vi "Alyssa_GlueFatLines.vi"(5 "Image Feed":T6=refnum, 7 "Template Path":path=path "C:/Users/Aerotech/Documents/BNL_ThermomechanicalStave/Utils/ConfigurationFiles_and_Templates/1_ModulePlacement", 8 "error in":errorcluster, 9 "um/pix resolution":dbl=1.58, 10 "Module corner coordinates":T2={"X [mm]"=-59.42477770816987, "Y [mm]"=4.341763392096446, "Z [mm] "=36.00000100000001}, 11 "XYZ Stage Control":refnum<k24>) -> (0 "error out":errorcluster={"status"=FALSE, "code"=1073676418, "source"="VISA Close in Alyssa_GlueFatLines.vi"}, 3 "XYZ .NET Refnum out":refnum<k24>)   [LabVIEW 2016]
uses:
  C:/Users/Aerotech/Documents/BNLStaveAssembly-blueprint/Bin/Aerotech.A3200.dll
  BNLStaveAssembly-blueprint/Bin/Aerotech.A3200.dll
  <vilib>/vision/Image Controls.llb/IMAQ Image.ctl
  <vilib>/LabVIEW Interface for Arduino/Type Defs/Arduino Resource.ctl
  <vilib>/LabVIEW Interface for Arduino/Type Defs/Board Type.ctl
  <vilib>/LabVIEW Interface for Arduino/Type Defs/Pin Mode.ctl
  <vilib>/Analysis/coordinate.llb/2D Cartesian Coordinate Rotation (Scalar).vi
  <vilib>/LabVIEW Interface for Arduino/LabVIEW Interface for Arduino.lvlib
  <vilib>/Analysis/NI_AALPro.lvlib
panel:
  in  "?":T1(tab)
  in  "Axis speeds (mm/s)":T3={"vX [mm]"=40.0, "vY [mm]"=40.0, "vZ [mm] "=40.0}
  in  "Home?":bool
  in  "Lowest Z Position":dbl=38.0
  out "Arduino Resource":T4={"VISA resource"="GlueCTRL", "Board Type"=enum."Uno", "Connection Type"=enum."USB / Serial", "Bytes Per Packet (15)"=15}
  in  "Digital I/O Pin":u8=7
  in  "Testing?":bool
  out "Difference camera/syringe in X":dbl=-133.03368290747076
  out "Difference camera/syringe in y":dbl=-2.170984960815403
  in  "Path to save collected images":path=path "C:/Users/Aerotech/cernbox/BNL/Stave Assembly Records/2017-06-12/3"
  in  "Estimate distance y":dbl
  in  "Estimate distance x":dbl=130.0
  in  "Lowest Z position Calibration":dbl=17.0
  in  "How many lines (actual x2)":i32=7
  in  "y dist (mm)":dbl=4.5
  out "bottom line speed":cluster{dbl, dbl, dbl}={32.78688524590164, 32.78688524590164, 32.78688524590164}
  out "mid line speed":cluster{dbl, dbl, dbl}={21.85792349726776, 21.85792349726776, 21.85792349726776}
  in  "Axial?":enum32{"Axial", "Right Stereo", "Left Stereo"}(radio)
  in  "glue time":dbl=1.83 format="%#_13g"
  out "top right speed":cluster{dbl, dbl, dbl}={5.46448087431694, 5.46448087431694, 5.46448087431694}
  out "top left speed":cluster{dbl, dbl, dbl}={21.85792349726776, 21.85792349726776, 21.85792349726776}
  out "Final Position":T7={"Final X"=-59.424942872475754, "Final Y"=8.342749448838399, "Final Z"=36.000300999844}
  out "Module Start":T7={"Final X"=-59.42477770816987, "Final Y"=4.341763392096446, "Final Z"=36.00000100000001}
  # "Overview: This takes a pattern of zeroes/ones (.csv file) as well as the start coordinates of the top left corner of a module and places dots of glue  \nRequirements: NI Arduino dependencies\nInstructions: Select a .csv file (ones indicate regions for glue) as well as a starting coordinate (this is default to the top left corner of the module spacer). You \ncan also input axis speeds (default to maximum) and module lengths and widths (default to 90 mm) which are the widths of the module to which you want to \nplace glue. Lastly, one can choose to Home the stage here and can select the lowest position in Z. The default is that the stage moves down 2-3 mm in Z \nwhile dispensing.  The Arduino inputs are default and simply allow the LabView program to drigger the Arduino (which sends a signal to the dispenser). The \nprogram signals to dispense air- all other parameters such as length of dispensing (default: 350 millisec), pressure (default: 48 psi), and vacuum pressure \n(default: 7.8 psi) are set on the dispenser itself. The defaults are highly recommended here."
  # "Positioning Inputs"
  # "Arduino Inputs"
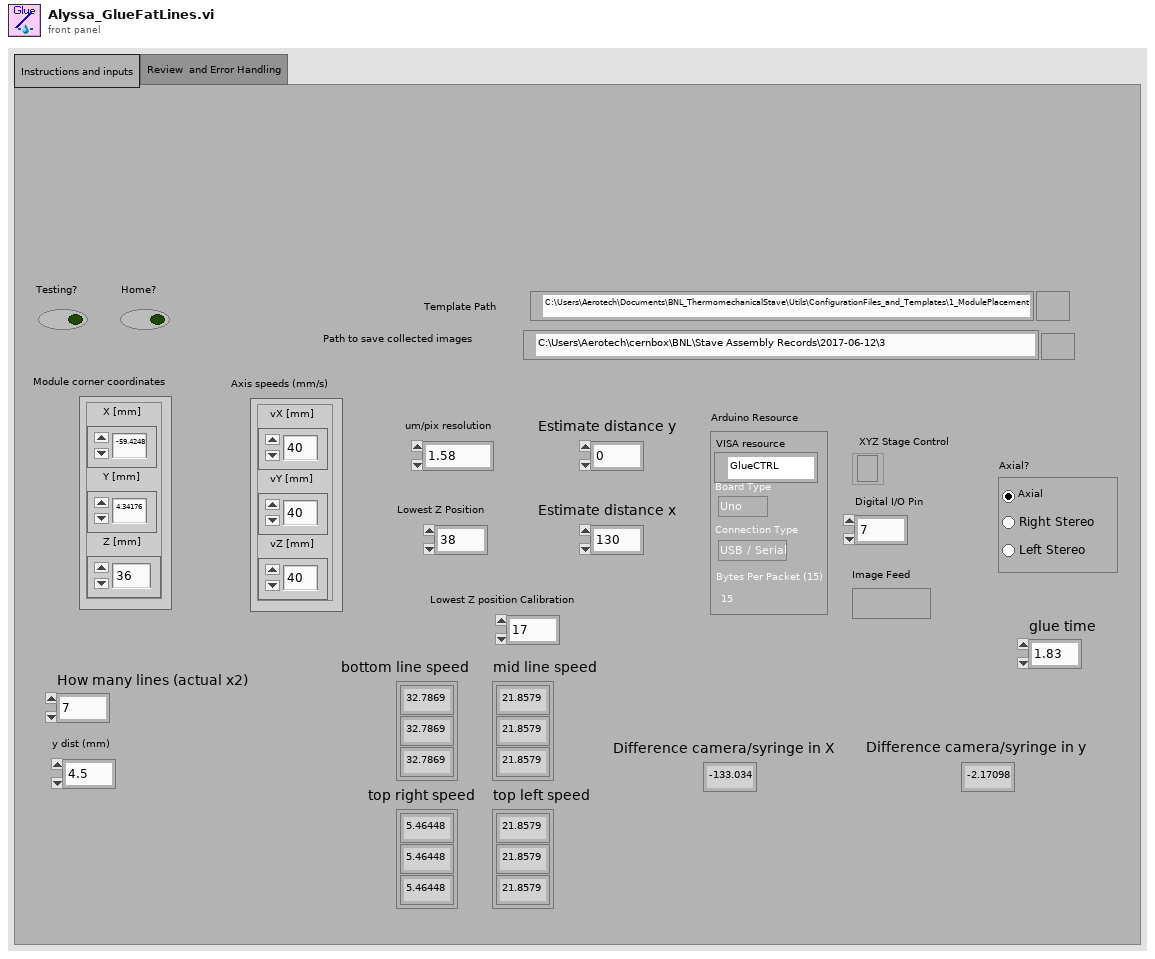
[diagram p1: front panel]
types:
  T1 = enum32{"Instructions and inputs", "Review  and Error Handling"}
  T2 = cluster{"X [mm]":dbl, "Y [mm]":dbl, "Z [mm] ":dbl}
  T3 = cluster{"vX [mm]":dbl, "vY [mm]":dbl, "vZ [mm] ":dbl}
  T4 = typedef "LabVIEW Interface for Arduino.lvlib/Arduino Resource.ctl" = cluster{"VISA resource":refnum<visa-resource-name>, "Board Type":T5, "Connection Type":enum8{"USB / Serial"}, "Bytes Per Packet (15)":u8}
  T5 = typedef "LabVIEW Interface for Arduino.lvlib/Board Type.ctl" = enum16{"Uno", "Dimuelanove w/Atmega 328", "Mega 2560"}
  T6 = typedef "IMAQ Image.ctl" = refnum<image>
  T7 = cluster{"Final X":dbl, "Final Y":dbl, "Final Z":dbl}
  T8 = typedef "LabVIEW Interface for Arduino.lvlib/Pin Mode.ctl" = enum8{"Input", "Output"}
  T9 = cluster{dbl, "Y [mm]":dbl, "Lowest Z Position":dbl}
  T10 = cluster{"Final X":dbl, "Final Y":dbl, "vZ [mm]":dbl}
  T11 = cluster{dbl, "Final Y":dbl, "Lowest Z Position":dbl}
  T12 = cluster{"Final X":dbl, "Final Y":dbl, "Z [mm] ":dbl}
  T13 = cluster{"x out":dbl, "y out":dbl, "Lowest Z Position":dbl}
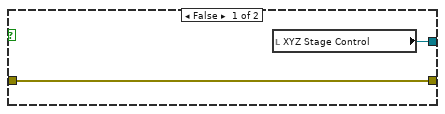
[diagram p2: hidden frame]
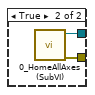
[diagram p3: hidden frame]
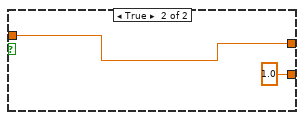
[diagram p5: hidden frame]
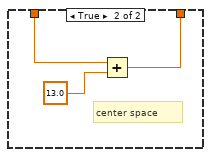
[diagram p6: hidden frame]
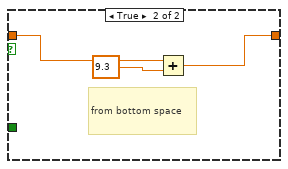
[diagram p7: hidden frame]
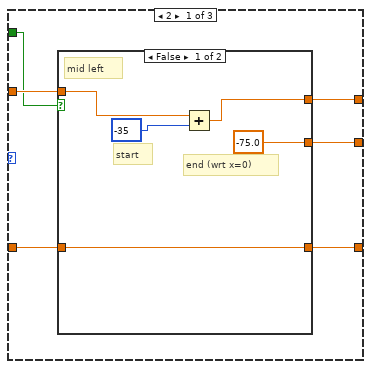
[diagram p8: hidden frame]
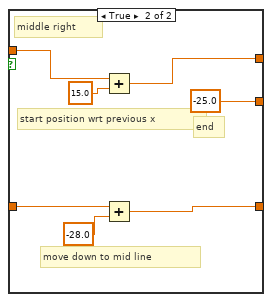
[diagram p9: hidden frame]
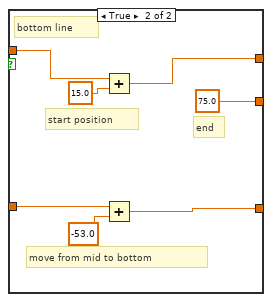
[diagram p10: hidden frame]
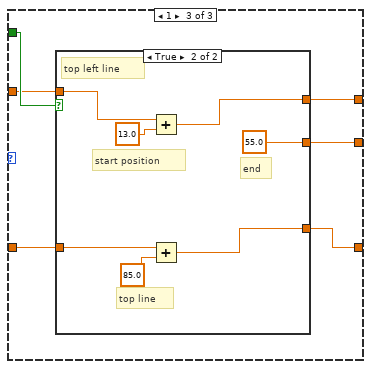
[diagram p11: hidden frame]
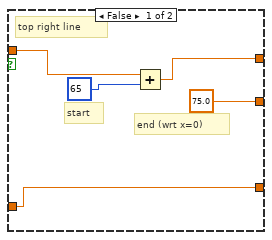
[diagram p12: hidden frame]
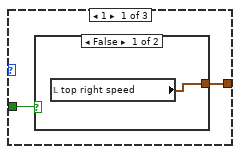
[diagram p13: hidden frame]
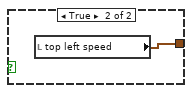
[diagram p14: hidden frame]
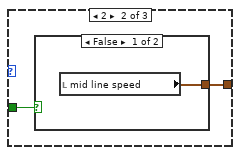
[diagram p15: hidden frame]
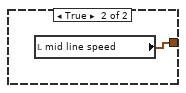
[diagram p16: hidden frame]
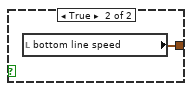
[diagram p17: hidden frame]
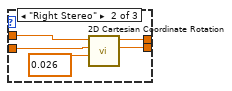
[diagram p18: hidden frame]
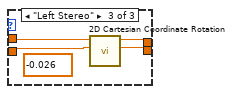
[diagram p19: hidden frame]
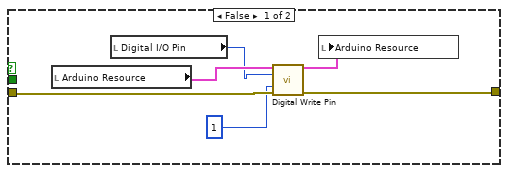
[diagram p20: hidden frame]
diagram:
  n1 = case shown="True" "Testing?" {
    tunnel: [w9 w11] -> w3
    tunnel: [w8 w10] -> w5
    tunnel: "error in" -> [w8 _]
    frame False {
      n2 = local read "XYZ Stage Control"() -> (w9:refnum<k24>)
    }
    frame True {
      n3 = case shown="False" "Home?" {
        tunnel: [w15 w21] -> w11
        tunnel: [w14 w20] -> w10
        frame False {
          w17 = string[] ["X", "Y", "Z"] ("Axes Names")
          n4 = call "Connect.vi"() -> ("error out"=w18:errorcluster, "controller"=w13:refnum<k24>)  [unwired: 10 in]
          n5 = call "EnableMultiple.vi"("error in (no error)"=w18, "axis names"=w17, "controller in"=w13) -> ("error out"=w19:errorcluster, "controller out"=w16:refnum<k24>)  [unwired: 7 in]
          n6 = call "GetCurrentXYZPosition (SubVI).vi"(".NET Refnum in - Device"=w16, "error in (no error)"=w19, "Axes Names"=w17) -> ("error out"=w14:errorcluster, ".NET Refnum out  - Device"=w15:refnum<k24>)  [unwired: 3 in, 4 out]
        }
        frame True {
          n7 = call "0_HomeAllAxes (SubVI).vi"() -> ("error out"=w20:errorcluster, "controller out"=w21:refnum<k24>)  [unwired: 8 in, 2 out]
        }
      }
    }
  }
  n8 = flat-sequence {
    tunnel: [w39] -> w7
    tunnel: w5 -> [w29]
    tunnel: w3 -> [w23]
    tunnel: [w192] -> w2
    tunnel: w7 -> [w195]
    tunnel: w2 -> [w347]
    tunnel: "Axial?" -> [w318]
    frame #0 {
      n9 = flat-sequence {
        tunnel: w29 -> [w53]
        tunnel: [w52] -> w24
        tunnel: w23 -> [w46]
        tunnel: w24 -> [w55]
        tunnel: [w54] -> w22
        tunnel: [w74] -> w26
        tunnel: w22 -> [w73]
        tunnel: w26 -> [w135]
        tunnel: [w133] -> w25
        tunnel: [w168] -> w27
        tunnel: w25 -> [w169]
        frame #0 {
          n10 = local read "Module corner coordinates"() -> (w48:T2)
          n11 = Unbundle(w48) -> ("X [mm]"=w45:dbl, "Y [mm]"=w42:dbl)  [unwired: 1 out]
          n12 = local read "Axis speeds (mm/s)"() -> (w51:T3)
          n13 = Add(x=w45, y=133.0) -> (x+y=w43:dbl)
          n14 = Bundle(w43, "Y [mm]"=w42, "Lowest Z Position"="Lowest Z Position") -> (w47:T9)  [unwired: 1 in]
          n15 = Bundle(w43, "Y [mm]"=w42, "Lowest Z Position"="Lowest Z Position") -> (w40:T9)  [unwired: 1 in]
          n16 = call "Go2XYZ (SubVI).vi"(".NET Refnum in"=w46, "Go to Coordinates"=w47, "Axis Speeds"=w51, "error in (no error)"=w53) -> (".NET Refnum out"=w50:refnum<k24>, "Final Position"=→"Final Position":T7, "error out"=w52:errorcluster)  [unwired: 7 in, 2 out]
          n17 = local write "Module corner coordinates"(w40) -> ()
          n18 = local write "XYZ Stage Control"(w50) -> ()
        }
        frame #1 {
          n19 = while {
            tunnel: w55 -> [w72]
            tunnel: [w68] -> w54
            stop <- w71 stop-if-true
            n20 = local read "Module corner coordinates"() -> (w66:T2)
            n21 = call "Lower glue mount"("error in (no error)"=w72) -> ("Move Z down"=w63:dbl, "Move Z up"=w62:dbl, "Accept current Z?"=w71:bool, "error out"=w69:errorcluster)  [unwired: 14 in, 1 out]
            n22 = local read "Lowest Z Position"() -> (w56:dbl)
            n23 = local read "Axis speeds (mm/s)"() -> (w70:T3)
            n24 = local read "XYZ Stage Control"() -> (w58:refnum<k24>)
            n25 = Add(x=w56, y=w63) -> (x+y=w60:dbl)
            n26 = Subtract(x=w60, y=w62) -> (x-y=w59:dbl)
            n27 = Unbundle(w66) -> ("X [mm]"=w65:dbl, "Y [mm]"=w64:dbl)  [unwired: 1 out]
            n28 = Bundle("X [mm]"=w65, "Y [mm]"=w64, w59) -> (w61:cluster{"X [mm]":dbl, "Y [mm]":dbl, dbl})  [unwired: 1 in]
            n29 = local write "Lowest Z Position"(w59) -> ()
            n30 = call "Go2XYZ (SubVI).vi"(".NET Refnum in"=w58, "Go to Coordinates"=w61, "Axis Speeds"=w70, "error in (no error)"=w69) -> (".NET Refnum out"=w67:refnum<k24>, "Final Position"=w57:T7, "error out"=w68:errorcluster)  [unwired: 7 in, 2 out]
            n31 = local write "XYZ Stage Control"(w67) -> ()
            n32 = local write "Final Position"(w57) -> ()
          }
        }
        frame #2 {
          n33 = call "Calibrate distance?"("error in (no error)"=w73) -> ("Calibrate distance?"=w75:bool, "error out"=w76:errorcluster)  [unwired: 16 in, 1 out]
          n34 = case shown="True" w75 {
            tunnel: w76 -> [w77 w79]
            tunnel: [w77 w80] -> w74
            frame False {
            }
            frame True {
              n35 = flat-sequence {
                tunnel: w79 -> [w82]
                tunnel: [w81] -> w78
                frame #0 {
                  n36 = local read "Final Position"() -> (w89:T7)
                  n37 = local read "Axis speeds (mm/s)"() -> (w85:T3)
                  n38 = local read "XYZ Stage Control"() -> (w84:refnum<k24>)
                  n39 = Unbundle(w89) -> ("Final X"=w87:dbl, "Final Y"=w88:dbl)  [unwired: 1 out]
                  n40 = Bundle("Final X"=w87, "Final Y"=w88, "vZ [mm]"=-20.0) -> (w91:T10)  [unwired: 1 in]
                  n41 = call "Go2XYZ (SubVI).vi"(".NET Refnum in"=w84, "Go to Coordinates"=w91, "Axis Speeds"=w85, "error in (no error)"=w82) -> (".NET Refnum out"=w83:refnum<k24>, "Final Position"=w86:T7, "error out"=w81:errorcluster)  [unwired: 7 in, 2 out]
                  n42 = local write "XYZ Stage Control"(w83) -> ()
                  n43 = local write "Final Position"(w86) -> ()
                }
              }
              n44 = while {
                tunnel: [w132] -> w80
                tunnel: w78 -> [w120]
                i -> [w117]
                stop <- w92 stop-if-true
                n45 = local read "Final Position"() -> (w94:T7)
                n46 = Unbundle(w94) -> ("Final X"=w99:dbl, "Final Y"=w97:dbl, "Final Z"=w98:dbl)
                n47 = local read "Testing?"() -> (w115:bool)
                n48 = local read "Axis speeds (mm/s)"() -> (w122:T3)
                n49 = local read "XYZ Stage Control"() -> (w118:refnum<k24>)
                n50 = Subtract(x=w97, y=220.0) -> (x-y=w95:dbl)
                n51 = Equal To 0?(x=w117) -> (x = 0?=w116:bool)
                n52 = And(x=w115, y=w116) -> (x .and. y?=w114:bool)
                n53 = Bundle("Final X"=w99, w95, "Final Z"=w98) -> (w100:cluster{"Final X":dbl, dbl, "Final Z":dbl})  [unwired: 1 in]
                n54 = call "CalibrateDistanceCameraSyringe.vi"("Path to save collected images"="Path to save collected images", "Image Feed"="Image Feed", "Off stave position"=w100, ".NET Refnum in"=w118, "Axis speeds (mm/s)"=w122, "Lowest Z Position"="Lowest Z position Calibration", "Estimate distance y"="Estimate distance y", "um/pix resolution"="um/pix resolution", "Estimate distance x"="Estimate distance x", "Template Path"="Template Path", "error in"=w120, "Testing?"=w114) -> ("XYZ .NET Refnum out"=w121:refnum<k24>, "error out"=w119:errorcluster, "X/Y difference (CAMERA - SYRINGE)"=w129:dbl[][])  [unwired: 1 in]
                n55 = local read "Difference camera/syringe in X"() -> (w104:dbl)
                n56 = local read "Difference camera/syringe in y"() -> (w101:dbl)
                n57 = local read "Lowest Z position Calibration"() -> (w106:dbl)
                n58 = call "Accept calibration?"("error in (no error)"=w119) -> ("Change in lowest Z"=w108:dbl, "Change in distance Y estimate"=w109:dbl, "Change in distance X estimate"=w110:dbl, "Accept the distance syringe/camera?"=w92:bool, "error out"=w132:errorcluster)  [unwired: 13 in, 1 out]
                n59 = local write "XYZ Stage Control"(w121) -> ()
                n60 = Index Array(array=w129, index (row) #1=0 ("index (row)"), index (col) #1=0 ("disabled index (col)"), index (row) #2=0 ("index (row)"), index (col) #2=1 ("disabled index (col)")) -> (element #1=→"Difference camera/syringe in X":dbl, element #2=→"Difference camera/syringe in y":dbl)
                n61 = Add(x=w104, y=w110) -> (x+y=w103:dbl)
                n62 = Add(x=w101, y=w109) -> (x+y=w102:dbl)
                n63 = Add(x=w106, y=w108) -> (x+y=w107:dbl)
                n64 = local write "Difference camera/syringe in X"(w103) -> ()
                n65 = local write "Difference camera/syringe in y"(w102) -> ()
                n66 = local write "Lowest Z position Calibration"(w107) -> ()
              }
            }
          }
        }
        frame #3 {
          n67 = flat-sequence {
            tunnel: w135 -> [w145]
            tunnel: [w142] -> w134
            tunnel: [w155] -> w133
            tunnel: w134 -> [w156]
            frame #0 {
              n68 = local read "Module corner coordinates"() -> (w154:T2)
              n69 = local read "Difference camera/syringe in y"() -> (w150:dbl)
              n70 = local read "Difference camera/syringe in X"() -> (w151:dbl)
              n71 = Unbundle By Name(w154) -> ("X [mm]"=w141:dbl, "Y [mm]"=w153:dbl)  [unwired: 1 out]
              n72 = Subtract(x=w153, y=w150) -> (x-y=w138:dbl)
              n73 = Subtract(x=w141, y=133.0) -> (x-y=w139:dbl)
              n74 = local read "Axis speeds (mm/s)"() -> (w146:T3)
              n75 = local read "XYZ Stage Control"() -> (w147:refnum<k24>)
              n76 = Subtract(x=w138, y=90.0) -> (x-y=w136:dbl)
              n77 = Subtract(x=w139, y=w151) -> (x-y=w152:dbl)
              n78 = Bundle(w152, w136, "index (row)"=-20.0) -> (w144:cluster{dbl, dbl, "index (row)":dbl})  [unwired: 1 in]
              n79 = call "Go2XYZ (SubVI).vi"(".NET Refnum in"=w147, "Go to Coordinates"=w144, "Axis Speeds"=w146, "error in (no error)"=w145) -> (".NET Refnum out"=w148:refnum<k24>, "Final Position"=w149:T7, "error out"=w142:errorcluster)  [unwired: 7 in, 2 out]
              n80 = local write "XYZ Stage Control"(w148) -> ()
              n81 = local write "Module corner coordinates"(w149) -> ()
            }
            frame #1 {
              n82 = local read "Module corner coordinates"() -> (w161:T2)
              n83 = local read "Lowest Z Position"() -> (w164:dbl)
              n84 = local read "Axis speeds (mm/s)"() -> (w158:T3)
              n85 = local read "XYZ Stage Control"() -> (w157:refnum<k24>)
              n86 = Unbundle(w161) -> ("X [mm]"=w162:dbl, "Y [mm]"=w163:dbl)  [unwired: 1 out]
              n87 = Subtract(x=w164, y=2.0) -> (x-y=w166:dbl)
              n88 = Bundle("X [mm]"=w162, "Y [mm]"=w163, w166) -> (w167:cluster{"X [mm]":dbl, "Y [mm]":dbl, dbl})  [unwired: 1 in]
              n89 = call "Go2XYZ (SubVI).vi"(".NET Refnum in"=w157, "Go to Coordinates"=w167, "Axis Speeds"=w158, "error in (no error)"=w156) -> (".NET Refnum out"=w159:refnum<k24>, "Final Position"=w160:T7, "error out"=w155:errorcluster)  [unwired: 7 in, 2 out]
              n90 = local write "XYZ Stage Control"(w159) -> ()
              n91 = local write "Module corner coordinates"(w160) -> ()
            }
          }
        }
        frame #4 {
          n92 = while {
            tunnel: w169 -> [w183]
            tunnel: [w185] -> w168
            stop <- w170 stop-if-true
            n93 = local read "Module corner coordinates"() -> (w182:T2)
            n94 = call "Ready to glue?"("error in (no error)"=w183) -> ("Move in Z"=w179:dbl, "Move in Y"=w180:dbl, "Move in X"=w181:dbl, "Oh yeah! Reset Arduino and go!"=w170:bool, "error out"=w184:errorcluster)  [unwired: 13 in, 1 out]
            n95 = local read "Axis speeds (mm/s)"() -> (w188:T3)
            n96 = local read "XYZ Stage Control"() -> (w186:refnum<k24>)
            n97 = Unbundle(w182) -> ("X [mm]"=w178:dbl, "Y [mm]"=w177:dbl, "Z [mm]"=w176:dbl)
            n98 = Add(x=w178, y=w181) -> (x+y=w173:dbl)
            n99 = Add(x=w177, y=w180) -> (x+y=w175:dbl)
            n100 = Add(x=w176, y=w179) -> (x+y=w174:dbl)
            n101 = Bundle(w173, w175, w174) -> (w172:cluster{dbl, dbl, dbl})  [unwired: 1 in]
            n102 = call "Go2XYZ (SubVI).vi"(".NET Refnum in"=w186, "Go to Coordinates"=w172, "Axis Speeds"=w188, "error in (no error)"=w184) -> (".NET Refnum out"=w187:refnum<k24>, "Final Position"=w171:T7, "error out"=w185:errorcluster)  [unwired: 7 in, 2 out]
            "Module Start" <- w171
            n103 = local write "XYZ Stage Control"(w187) -> ()
            n104 = local write "Final Position"(w171) -> ()
            n105 = local write "Module corner coordinates"(w171) -> ()
          }
        }
      }
      n106 = local read "Digital I/O Pin"() -> (w28:u8)
      n107 = call <vilib>:"Init.vi"("VISA resource"=refnum<visa-resource-name> "GlueCTRL", "error in"=w27) -> ("Arduino Resource"=w31:T4, "error out"=w32:errorcluster)  [unwired: 16 in]
      "Arduino Resource" <- w31
      n108 = call <vilib>:"Set Digital Pin Mode.vi"("Arduino Resource"=w31, "Digital I/O Pin"="Digital I/O Pin", "Pin Mode (Input)"=Pin_Mode."Output", "error in"=w32) -> ("Arduino Resource"=w35:T4, "error out"=w36:errorcluster)  [unwired: 10 in]
      n109 = call <vilib>:"Digital Write Pin.vi"("Arduino Resource"=w35, "Digital I/O Pin (0)"=w28, "Value (0)"=u8 0, "error in"=w36) -> ("Arduino Resource"=w30:T4, "error out"=w39:errorcluster)  [unwired: 10 in]
      n110 = local write "Arduino Resource"(w30) -> ()
    }
    frame #1 {
      n111 = local read "Module Start"() -> (w194:T7)
      n112 = Unbundle By Name(w194) -> ("Final X"=w189:dbl, "Final Y"=w190:dbl, "Final Z"=w193:dbl)
      n113 = for {
        N: "How many lines (actual x2)" -> [_]
        tunnel: w195 -> [w209]
        tunnel: [w208] -> w192
        shift-right: [w207] -> _
        shift-left: w190 -> [w196]
        tunnel: w193 -> [w206]
        shift-right: [w205] -> _
        shift-left: w189 -> [w197]
        i -> [w200]
        n114 = local read "How many lines (actual x2)"() -> (w203:i32)
        n115 = Subtract(x=w203, y=2) -> (x-y=w201:i32)
        n116 = Equal?(x=w200, y=w201) -> (x = y?=w198:bool)
        n117 = Equal To 0?(x=w200) -> (x = 0?=w199:bool)
        n118 = for {
          N: 2 -> [_]
          tunnel: w209 -> [w231]
          tunnel: [w229] -> w208
          shift-right: [w228] -> w207
          shift-left: w196 -> [w219]
          tunnel: w206 -> [w218]
          tunnel: w197 -> [w220]
          tunnel: [w216] -> w205
          tunnel: w199 -> [w211]
          tunnel: w198 -> [w210]
          i -> [w217]
          n119 = flat-sequence {
            tunnel: w231 -> [w249]
            tunnel: [w234] -> w226
            tunnel: [w249] -> w225
            tunnel: [w237] -> w224
            tunnel: [w236] -> w223
            tunnel: [w248] -> w222
            tunnel: [w237] -> w221
            tunnel: w220 -> [w235]
            tunnel: w219 -> [w238]
            tunnel: w218 -> [w248]
            tunnel: w217 -> [w242]
            tunnel: w211 -> [w241]
            tunnel: w210 -> [w240]
            tunnel: [w277] -> w214
            tunnel: [w278] -> w213
            tunnel: [w279] -> w212
            tunnel: w221 -> [w279]
            tunnel: w222 -> [w276]
            tunnel: w223 -> [w269]
            tunnel: w224 -> [w268]
            tunnel: w225 -> [w272]
            tunnel: w226 -> [w277]
            tunnel: [w297] -> w233
            tunnel: [w296] -> w232
            tunnel: [w295] -> w230
            tunnel: [w288] -> w227
            tunnel: w214 -> [w285]
            tunnel: w213 -> [w287]
            tunnel: w212 -> [w288]
            tunnel: [w285] -> w215
            tunnel: [w317] -> w229
            tunnel: w230 -> [w305]
            tunnel: w232 -> [w316]
            tunnel: w233 -> [w314]
            tunnel: [w304] -> w228
            tunnel: w227 -> [w304]
            tunnel: [w303] -> w216
            tunnel: w215 -> [w303]
            frame #0 {
              # "line length"
              n120 = Equal To 0?(x=w242) -> (x = 0?=w239:bool)
              n121 = And(x=w239, y=w241) -> (x .and. y?=w243:bool)
              n122 = And(x=w239, y=w240) -> (x .and. y?=w247:bool)
              n123 = case shown="False" w239 {
                tunnel: [0.0 1.0] -> w244
                tunnel: [w251 w254] -> w236
                tunnel: w235 -> [w252 w254]
                frame False {
                  # "start @ end of line"
                  n124 = Add(x=w252, y=90 ("x")) -> (x+y=w251:dbl)
                }
                frame True {
                }
              }
              n125 = case shown="False" w243 {
                tunnel: w238 -> [w257 w267]
                tunnel: [w258 w266] -> w237
                tunnel: w247 -> [w256 _]
                frame False {
                  n126 = case shown="False" w256 {
                    tunnel: [w261 w262] -> w258
                    tunnel: w257 -> [w259 w264]
                    frame False {
                      n127 = Add(x=w259, y="y dist (mm)") -> (x+y=w261:dbl)
                    }
                    frame True {
                      # "center space"
                      n128 = Add(x=w264, y=13.0) -> (x+y=w262:dbl)
                    }
                  }
                }
                frame True {
                  # "from bottom space"
                  n129 = Add(x=w267, y=9.3) -> (x+y=w266:dbl)
                }
              }
              n130 = Multiply(x=90, y=w244) -> (x*y=w245:dbl)
              n131 = Add(x=w235, y=w245) -> (x+y=w234:dbl)
            }
            frame #1 {
              n132 = local read "XYZ Stage Control"() -> (w271:refnum<k24>)
              n133 = local read "Axis speeds (mm/s)"() -> (w274:T3)
              n134 = Bundle("Final X"=w269, w268, "Final Z"=w276) -> (w275:cluster{"Final X":dbl, dbl, "Final Z":dbl})  [unwired: 1 in]
              n135 = call "Go2XYZ (SubVI).vi"(".NET Refnum in"=w271, "Go to Coordinates"=w275, "Axis Speeds"=w274, "error in (no error)"=w272) -> (".NET Refnum out"=w270:refnum<k24>, "Final Position"=w273:T7, "error out"=w278:errorcluster)  [unwired: 7 in, 2 out]
              n136 = local write "XYZ Stage Control"(w270) -> ()
              n137 = local write "Final Position"(w273) -> ()
            }
            frame #2 {
              n138 = local read "Final Position"() -> (w289:T7)
              n139 = local read "Lowest Z Position"() -> (w294:dbl)
              n140 = local read "Axis speeds (mm/s)"() -> (w284:T3)
              n141 = local read "Arduino Resource"() -> (w298:T4)
              n142 = local read "Digital I/O Pin"() -> (w297:u8)
              n143 = local read "XYZ Stage Control"() -> (w292:refnum<k24>)
              n144 = Unbundle(w289) -> ("Final Y"=w286:dbl)  [unwired: 2 out]
              n145 = Unbundle(w284) -> ("vX [mm]"=w283:dbl, "vZ [mm]"=w282:dbl)  [unwired: 1 out]
              n146 = Bundle(w285, "Final Y"=w286, "Lowest Z Position"=w294) -> (w291:T11)  [unwired: 1 in]
              n147 = Bundle("vX [mm]"=w283, "x"=1.04, "vZ [mm]"=w282) -> (w281:cluster{"vX [mm]":dbl, "x":dbl, "vZ [mm] ":dbl})  [unwired: 1 in]
              n148 = call <vilib>:"Digital Write Pin.vi"("Arduino Resource"=w298, "Digital I/O Pin (0)"=w297, "Value (0)"=u8 1, "error in"=w287) -> ("Arduino Resource"=w296:T4, "error out"=w295:errorcluster)  [unwired: 10 in]
              n149 = call "Go2XYZ (SubVI).vi"(".NET Refnum in"=w292, "Go to Coordinates"=w291, "Axis Speeds"=w281) -> (".NET Refnum out"=w293:refnum<k24>, "Final Position"=w290:T7)  [unwired: 8 in, 3 out]
              n150 = local write "Arduino Resource"(w296) -> ()
              n151 = local write "XYZ Stage Control"(w293) -> ()
              n152 = local write "Final Position"(w290) -> ()
            }
            frame #3 {
              n153 = local read "Final Position"() -> (w312:T7)
              n154 = local read "Module corner coordinates"() -> (w311:T2)
              n155 = call <vilib>:"Digital Write Pin.vi"("Arduino Resource"=w316, "Digital I/O Pin (0)"=w314, "Value (0)"=u8 0, "error in"=w305) -> ("Arduino Resource"=w313:T4, "error out"=w317:errorcluster)  [unwired: 10 in]
              n156 = local write "Arduino Resource"(w313) -> ()
              n157 = Unbundle(w312) -> ("Final X"=w302:dbl, "Final Y"=w301:dbl)  [unwired: 1 out]
              n158 = local read "XYZ Stage Control"() -> (w307:refnum<k24>)
              n159 = local read "Axis speeds (mm/s)"() -> (w308:T3)
              n160 = Unbundle(w311) -> ("Z [mm]"=w310:dbl)  [unwired: 2 out]
              n161 = Bundle("Final X"=w302, "Final Y"=w301, "Z [mm]"=w310) -> (w309:T12)  [unwired: 1 in]
              n162 = call "Go2XYZ (SubVI).vi"(".NET Refnum in"=w307, "Go to Coordinates"=w309, "Axis Speeds"=w308) -> (".NET Refnum out"=w300:refnum<k24>, "Final Position"=w306:T7)  [unwired: 8 in, 3 out]
              n163 = local write "Final Position"(w306) -> ()
              n164 = local write "XYZ Stage Control"(w300) -> ()
            }
          }
        }
      }
    }
    frame #2 {
      n165 = local read "glue time"() -> (w332:dbl)
      n166 = local read "Module Start"() -> (w348:T7)
      n167 = Unbundle By Name(w348) -> ("Final X"=w336:dbl, "Final Y"=w337:dbl, "Final Z"=w346:dbl)
      n168 = Divide(x=40.0 ("vX [mm]"), y=w332) -> (x/y=w330:dbl)
      n169 = Divide(x=60.0 ("vX [mm]"), y="glue time") -> (x/y=w331:dbl)
      n170 = Bundle(w330, w330, w330) -> (→"mid line speed":cluster{dbl, dbl, dbl})  [unwired: 1 in]
      n171 = Bundle(w331, w331, w331) -> (→"bottom line speed":cluster{dbl, dbl, dbl})  [unwired: 1 in]
      n172 = for {
        N: 3 -> [_]
        tunnel: w347 -> [w366]
        tunnel: [w365] -> w340
        shift-right: [w363] -> _
        shift-left: w337 -> [w364]
        tunnel: w346 -> [w362]
        shift-right: [w361] -> _
        shift-left: w336 -> [w360]
        tunnel: w318 -> [w351]
        tunnel: w318 -> [w350]
        tunnel: w318 -> [w349]
        i -> [w355]
        n173 = Equal?(x=w355, y=2) -> (x = y?=w352:bool)
        n174 = Equal?(x=w355, y=1) -> (x = y?=w353:bool)
        n175 = Equal?(x=w355, y=0) -> (x = y?=w354:bool)
        n176 = for {
          N: 2 -> [_]
          tunnel: w366 -> [w401]
          tunnel: [w399] -> w365
          shift-right: [w398] -> w363
          shift-left: w364 -> [w390]
          tunnel: w362 -> [w389]
          tunnel: w360 -> [w382]
          tunnel: [w387] -> w361
          tunnel: w354 -> [w381]
          tunnel: w353 -> [w380]
          tunnel: w352 -> [w371]
          tunnel: w351 -> [w369]
          tunnel: w350 -> [w368]
          tunnel: w349 -> [w367]
          i -> [w388]
          n177 = flat-sequence {
            tunnel: w401 -> [w416]
            tunnel: [w414] -> w396
            tunnel: [w416] -> w395
            tunnel: [w406] -> w394
            tunnel: [w407] -> w393
            tunnel: [w415] -> w392
            tunnel: [w406] -> w391
            tunnel: w382 -> [w405]
            tunnel: w390 -> [w404]
            tunnel: w389 -> [w415]
            tunnel: w388 -> [w412]
            tunnel: w381 -> [w411]
            tunnel: w380 -> [w410]
            tunnel: w371 -> [w409]
            tunnel: [w403] -> w379
            tunnel: [w402] -> w378
            tunnel: [w402] -> w372
            tunnel: [w486] -> w385
            tunnel: [w485] -> w384
            tunnel: [w484] -> w383
            tunnel: w391 -> [w484]
            tunnel: w392 -> [w483]
            tunnel: w393 -> [w477]
            tunnel: w394 -> [w476]
            tunnel: w395 -> [w480]
            tunnel: w396 -> [w486]
            tunnel: w379 -> [w472]
            tunnel: w378 -> [w471]
            tunnel: [w472] -> w377
            tunnel: [w471] -> w376
            tunnel: [w470] -> w373
            tunnel: w372 -> [w470]
            tunnel: w369 -> [w469]
            tunnel: [w528] -> w400
            tunnel: [w521] -> w397
            tunnel: w385 -> [w519]
            tunnel: w384 -> [w520]
            tunnel: w383 -> [w521]
            tunnel: [w519] -> w386
            tunnel: w377 -> [w514]
            tunnel: w376 -> [w513]
            tunnel: [w514] -> w375
            tunnel: [w513] -> w374
            tunnel: w371 -> [w512]
            tunnel: w373 -> [w511]
            tunnel: [w511] -> w370
            tunnel: w368 -> [w510]
            tunnel: [w588] -> w399
            tunnel: w400 -> [w581]
            tunnel: [w580] -> w398
            tunnel: w397 -> [w580]
            tunnel: [w579] -> w387
            tunnel: w386 -> [w579]
            tunnel: w375 -> [w573]
            tunnel: w374 -> [w572]
            tunnel: w371 -> [w571]
            tunnel: w370 -> [w570]
            tunnel: w367 -> [w569]
            frame #0 {
              # "where to move"
              n178 = Build Array(w411, w410, w409) -> (w413:bool[])
              n179 = Equal To 0?(x=w412) -> (x = 0?=w402:bool)
              n180 = Boolean Array To Number(Boolean array=w413) -> (number=w403:u32)
              n181 = case shown="0, Default" w403 {
                tunnel: w402 -> [w417 w436 w456]
                tunnel: w405 -> [w421 w435 w455]
                tunnel: w404 -> [w422 w440 w454]
                tunnel: [w420 w437 w453] -> w406
                tunnel: [w419 w438 w452] -> w408
                tunnel: [w418 w439 w451] -> w407
                frame 2 {
                  n182 = case shown="False" w417 {
                    tunnel: [w426 w433] -> w418
                    tunnel: w421 -> [w427 w434]
                    tunnel: [-75.0 -25.0 ("y")] -> w419
                    tunnel: w422 -> [w423 w429]
                    tunnel: [w423 w428] -> w420
                    frame False {
                      # "mid left"
                      # "end (wrt x=0)"
                      # "start"
                      n183 = Add(x=w427, y=-35 ("x")) -> (x+y=w426:dbl)
                    }
                    frame True {
                      # "move down to mid line"
                      # "end"
                      # "middle right"
                      # "start position wrt previous x"
                      n184 = Add(x=w434, y=15.0) -> (x+y=w433:dbl)
                      n185 = Add(x=w429, y=-28.0) -> (x+y=w428:dbl)
                    }
                  }
                }
                frame 0, Default {
                  n186 = case shown="False" w436 {
                    tunnel: [w442 w449] -> w439
                    tunnel: w435 -> [w442 w450]
                    tunnel: [0.0 ("y") 75.0 ("y")] -> w438
                    tunnel: w440 -> [w443 w445]
                    tunnel: [w443 w444] -> w437
                    frame False {
                      # "do nothing"
                    }
                    frame True {
                      # "move from mid to bottom"
                      # "end"
                      # "bottom line"
                      # "start position"
                      n187 = Add(x=w450, y=15.0) -> (x+y=w449:dbl)
                      n188 = Add(x=w445, y=-53.0) -> (x+y=w444:dbl)
                    }
                  }
                }
                frame 1 {
                  n189 = case shown="True" w456 {
                    tunnel: [w460 w467] -> w451
                    tunnel: w455 -> [w461 w468]
                    tunnel: [75.0 55.0 ("y")] -> w452
                    tunnel: w454 -> [w457 w463]
                    tunnel: [w457 w462] -> w453
                    frame False {
                      # "top right line"
                      # "end (wrt x=0)"
                      # "start"
                      n190 = Add(x=w461, y=65 ("x")) -> (x+y=w460:dbl)
                    }
                    frame True {
                      # "top line"
                      # "end"
                      # "top left line"
                      # "start position"
                      n191 = Add(x=w468, y=13.0) -> (x+y=w467:dbl)
                      n192 = Add(x=w463, y=85.0) -> (x+y=w462:dbl)
                    }
                  }
                }
              }
              n193 = Add(x=w405, y=w408) -> (x+y=w414:dbl)
            }
            frame #1 {
              n194 = case shown="0, Default" w472 {
                tunnel: w471 -> [w488 w492 w496]
                tunnel: [w487 w491 w495] -> w473
                frame 1 {
                  n195 = case shown="False" w488 {
                    tunnel: [w489 w490] -> w487
                    frame False {
                      n196 = local read "top right speed"() -> (w489:cluster{dbl, dbl, dbl})
                    }
                    frame True {
                      n197 = local read "top left speed"() -> (w490:cluster{dbl, dbl, dbl})
                    }
                  }
                }
                frame 2 {
                  n198 = case shown="False" w492 {
                    tunnel: [w493 w494] -> w491
                    frame False {
                      n199 = local read "mid line speed"() -> (w493:cluster{dbl, dbl, dbl})
                    }
                    frame True {
                      n200 = local read "mid line speed"() -> (w494:cluster{dbl, dbl, dbl})
                    }
                  }
                }
                frame 0, Default {
                  n201 = case shown="False" w496 {
                    tunnel: [w497 w498] -> w495
                    frame False {
                      n202 = local read "bottom line speed"() -> (w497:cluster{dbl, dbl, dbl})
                    }
                    frame True {
                      n203 = local read "bottom line speed"() -> (w498:cluster{dbl, dbl, dbl})
                    }
                  }
                }
              }
              n204 = case shown="\"Axial\", Default" w469 {
                tunnel: w477 -> [w500 w505 w507]
                tunnel: w476 -> [w499 w504 w506]
                tunnel: [w500 w502 w509] -> w475
                tunnel: [w499 w501 w508] -> w474
                frame "Axial", Default {
                }
                frame "Right Stereo" {
                  n205 = call-poly <vilib>:"2D Cartesian Coordinate Rotation.vi"("theta"=0.026, "y"=w504, "x"=w505) -> ("y out"=w501:dbl, "x out"=w502:dbl)  [unwired: 6 in, 1 out]
                }
                frame "Left Stereo" {
                  (unwired) -0.026 ("theta")
                  n206 = call-poly <vilib>:"2D Cartesian Coordinate Rotation.vi"("y"=w506, "x"=w507) -> ("y out"=w508:dbl, "x out"=w509:dbl)  [unwired: 7 in, 1 out]
                }
              }
              n207 = Bundle("x out"=w475, "y out"=w474, "Final Z"=w483) -> (w482:cluster{"x out":dbl, "y out":dbl, "Final Z":dbl})  [unwired: 1 in]
              n208 = local read "XYZ Stage Control"() -> (w479:refnum<k24>)
              n209 = call "Go2XYZ (SubVI).vi"(".NET Refnum in"=w479, "Go to Coordinates"=w482, "Axis Speeds"=w473, "error in (no error)"=w480) -> (".NET Refnum out"=w478:refnum<k24>, "Final Position"=w481:T7, "error out"=w485:errorcluster)  [unwired: 7 in, 2 out]
              n210 = local write "Final Position"(w481) -> ()
              n211 = local write "XYZ Stage Control"(w478) -> ()
            }
            frame #2 {
              n212 = local read "Final Position"() -> (w522:T7)
              n213 = case shown="True" w512 {
                tunnel: [w531 w537] -> w528
                tunnel: w520 -> [w530 w536]
                tunnel: w511 -> [_ w535]
                frame False {
                  n214 = local read "Arduino Resource"() -> (w534:T4)
                  n215 = local read "Digital I/O Pin"() -> (w533:u8)
                  n216 = call <vilib>:"Digital Write Pin.vi"("Arduino Resource"=w534, "Digital I/O Pin (0)"=w533, "Value (0)"=u8 1, "error in"=w530) -> ("Arduino Resource"=w532:T4, "error out"=w531:errorcluster)  [unwired: 10 in]
                  n217 = local write "Arduino Resource"(w532) -> ()
                }
                frame True {
                  n218 = case shown="True" w535 {
                    tunnel: [w538 w540] -> w537
                    tunnel: w536 -> [w538 w539]
                    frame False {
                    }
                    frame True {
                      n219 = local read "Arduino Resource"() -> (w543:T4)
                      n220 = local read "Digital I/O Pin"() -> (w542:u8)
                      n221 = call <vilib>:"Digital Write Pin.vi"("Arduino Resource"=w543, "Digital I/O Pin (0)"=w542, "Value (0)"=u8 1, "error in"=w539) -> ("Arduino Resource"=w541:T4, "error out"=w540:errorcluster)  [unwired: 10 in]
                      n222 = local write "Arduino Resource"(w541) -> ()
                    }
                  }
                }
              }
              n223 = Unbundle(w522) -> ("Final Y"=w518:dbl)  [unwired: 2 out]
              n224 = case shown="2" w514 {
                tunnel: w513 -> [w546 w550 w554]
                tunnel: [w545 w549 w553] -> w515
                frame 1 {
                  n225 = case shown="False" w546 {
                    tunnel: [w547 w548] -> w545
                    frame False {
                      n226 = local read "top right speed"() -> (w547:cluster{dbl, dbl, dbl})
                    }
                    frame True {
                      n227 = local read "top left speed"() -> (w548:cluster{dbl, dbl, dbl})
                    }
                  }
                }
                frame 2 {
                  n228 = case shown="False" w550 {
                    tunnel: [w551 w552] -> w549
                    frame False {
                      n229 = local read "mid line speed"() -> (w551:cluster{dbl, dbl, dbl})
                    }
                    frame True {
                      n230 = local read "mid line speed"() -> (w552:cluster{dbl, dbl, dbl})
                    }
                  }
                }
                frame 0, Default {
                  n231 = case shown="False" w554 {
                    tunnel: [w555 w556] -> w553
                    frame False {
                      n232 = local read "bottom line speed"() -> (w555:cluster{dbl, dbl, dbl})
                    }
                    frame True {
                      n233 = local read "bottom line speed"() -> (w556:cluster{dbl, dbl, dbl})
                    }
                  }
                }
              }
              n234 = local read "Lowest Z Position"() -> (w527:dbl)
              n235 = case shown="\"Axial\", Default" w510 {
                tunnel: w519 -> [w558 w563 w565]
                tunnel: w518 -> [w557 w562 w564]
                tunnel: [w558 w560 w567] -> w516
                tunnel: [w557 w559 w566] -> w517
                frame "Axial", Default {
                }
                frame "Right Stereo" {
                  n236 = call-poly <vilib>:"2D Cartesian Coordinate Rotation.vi"("theta"=0.026, "y"=w562, "x"=w563) -> ("y out"=w559:dbl, "x out"=w560:dbl)  [unwired: 6 in, 1 out]
                }
                frame "Left Stereo" {
                  (unwired) -0.026 ("theta")
                  n237 = call-poly <vilib>:"2D Cartesian Coordinate Rotation.vi"("y"=w564, "x"=w565) -> ("y out"=w566:dbl, "x out"=w567:dbl)  [unwired: 7 in, 1 out]
                }
              }
              n238 = local read "XYZ Stage Control"() -> (w525:refnum<k24>)
              n239 = Bundle("x out"=w516, "y out"=w517, "Lowest Z Position"=w527) -> (w524:T13)  [unwired: 1 in]
              n240 = call "Go2XYZ (SubVI).vi"(".NET Refnum in"=w525, "Go to Coordinates"=w524, "Axis Speeds"=w515) -> (".NET Refnum out"=w526:refnum<k24>, "Final Position"=w523:T7)  [unwired: 8 in, 3 out]
              n241 = local write "XYZ Stage Control"(w526) -> ()
              n242 = local write "Final Position"(w523) -> ()
            }
            frame #3 {
              n243 = local read "Final Position"() -> (w587:T7)
              n244 = case shown="True" w571 {
                tunnel: [w590 w597] -> w588
                tunnel: w581 -> [w589 w596]
                tunnel: w570 -> [_ w595]
                frame False {
                  n245 = local read "Digital I/O Pin"() -> (w591:u8)
                  n246 = local read "Arduino Resource"() -> (w592:T4)
                  n247 = call <vilib>:"Digital Write Pin.vi"("Arduino Resource"=w592, "Digital I/O Pin (0)"=w591, "Value (0)"=u8 0, "error in"=w589) -> ("Arduino Resource"=w593:T4, "error out"=w590:errorcluster)  [unwired: 10 in]
                  n248 = local write "Arduino Resource"(w593) -> ()
                }
                frame True {
                  n249 = case shown="True" w595 {
                    tunnel: [w598 w604] -> w597
                    tunnel: w596 -> [w598 w601]
                    frame False {
                    }
                    frame True {
                      n250 = local read "Digital I/O Pin"() -> (w599:u8)
                      n251 = local read "Arduino Resource"() -> (w600:T4)
                      n252 = call <vilib>:"Digital Write Pin.vi"("Arduino Resource"=w600, "Digital I/O Pin (0)"=w599, "Value (0)"=u8 0, "error in"=w601) -> ("Arduino Resource"=w602:T4, "error out"=w604:errorcluster)  [unwired: 10 in]
                      n253 = local write "Arduino Resource"(w602) -> ()
                    }
                  }
                }
              }
              n254 = local read "Module Start"() -> (w586:T7)
              n255 = Unbundle(w587) -> ("Final X"=w577:dbl, "Final Y"=w578:dbl)  [unwired: 1 out]
              n256 = Unbundle(w586) -> ("Final Z"=w585:dbl)  [unwired: 2 out]
              n257 = case shown="\"Axial\", Default" w569 {
                tunnel: w577 -> [w618 w623 w625]
                tunnel: w578 -> [w617 w622 w624]
                tunnel: [w618 w620 w627] -> w576
                tunnel: [w617 w619 w626] -> w575
                frame "Axial", Default {
                }
                frame "Right Stereo" {
                  n258 = call-poly <vilib>:"2D Cartesian Coordinate Rotation.vi"("theta"=0.026, "y"=w622, "x"=w623) -> ("y out"=w619:dbl, "x out"=w620:dbl)  [unwired: 6 in, 1 out]
                }
                frame "Left Stereo" {
                  (unwired) -0.026 ("theta")
                  n259 = call-poly <vilib>:"2D Cartesian Coordinate Rotation.vi"("y"=w624, "x"=w625) -> ("y out"=w626:dbl, "x out"=w627:dbl)  [unwired: 7 in, 1 out]
                }
              }
              n260 = local read "XYZ Stage Control"() -> (w583:refnum<k24>)
              n261 = case shown="0, Default" w573 {
                tunnel: w572 -> [w606 w610 w614]
                tunnel: [w605 w609 w613] -> w574
                frame 1 {
                  n262 = case shown="False" w606 {
                    tunnel: [w607 w608] -> w605
                    frame False {
                      n263 = local read "top right speed"() -> (w607:cluster{dbl, dbl, dbl})
                    }
                    frame True {
                      n264 = local read "top left speed"() -> (w608:cluster{dbl, dbl, dbl})
                    }
                  }
                }
                frame 2 {
                  n265 = case shown="False" w610 {
                    tunnel: [w611 w612] -> w609
                    frame False {
                      n266 = local read "mid line speed"() -> (w611:cluster{dbl, dbl, dbl})
                    }
                    frame True {
                      n267 = local read "mid line speed"() -> (w612:cluster{dbl, dbl, dbl})
                    }
                  }
                }
                frame 0, Default {
                  n268 = case shown="False" w614 {
                    tunnel: [w615 w616] -> w613
                    frame False {
                      n269 = local read "bottom line speed"() -> (w615:cluster{dbl, dbl, dbl})
                    }
                    frame True {
                      n270 = local read "bottom line speed"() -> (w616:cluster{dbl, dbl, dbl})
                    }
                  }
                }
              }
              n271 = Bundle("x out"=w576, "y out"=w575, "Final Z"=w585) -> (w584:cluster{"x out":dbl, "y out":dbl, "Final Z":dbl})  [unwired: 1 in]
              n272 = call "Go2XYZ (SubVI).vi"(".NET Refnum in"=w583, "Go to Coordinates"=w584, "Axis Speeds"=w574) -> (".NET Refnum out"=→"XYZ .NET Refnum out":refnum<k24>, "Final Position"=w582:T7)  [unwired: 8 in, 3 out]
              n273 = local write "Final Position"(w582) -> ()
            }
          }
        }
      }
      n274 = local read "glue time"() -> (w320:dbl)
      n275 = local read "glue time"() -> (w324:dbl)
      n276 = Divide(x=10.0 ("vX [mm]"), y=w320) -> (x/y=w321:dbl)
      n277 = Divide(x=40.0 ("vX [mm]"), y=w324) -> (x/y=w325:dbl)
      n278 = Bundle(w321, w321, w321) -> (→"top right speed":cluster{dbl, dbl, dbl})  [unwired: 1 in]
      n279 = Bundle(w325, w325, w325) -> (→"top left speed":cluster{dbl, dbl, dbl})  [unwired: 1 in]
      n280 = local read "Arduino Resource"() -> (w339:T4)
      n281 = local read "Digital I/O Pin"() -> (w338:u8)
      n282 = call <vilib>:"Digital Write Pin.vi"("Arduino Resource"=w339, "Digital I/O Pin (0)"=w338, "error in"=w340) -> ("Arduino Resource"=w344:T4, "error out"=w343:errorcluster)  [unwired: 11 in]
      n283 = call <vilib>:"Close.vi"("Arduino Resource"=w344, "error in"=w343) -> ("error out"=w342:errorcluster)  [unwired: 13 in]
      n284 = VISA Close(VISA resource name=refnum<visa-resource-name> "GlueCTRL", error in (no error)=w342) -> (error out=→"error out":errorcluster)
    }
  }
